vi "CRYO_MASTER_FULL_RUN2.vi"() -> ()   [LabVIEW 2017] (continued)
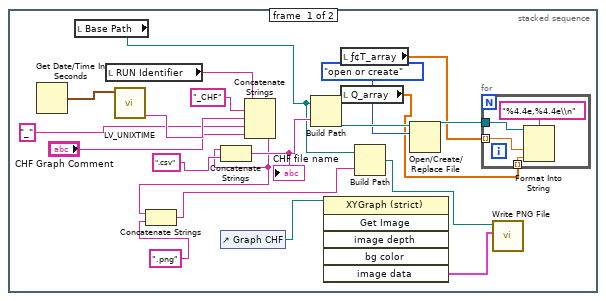
[diagram p3: hidden frame]
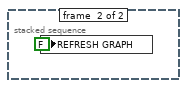
[diagram p5: hidden frame]
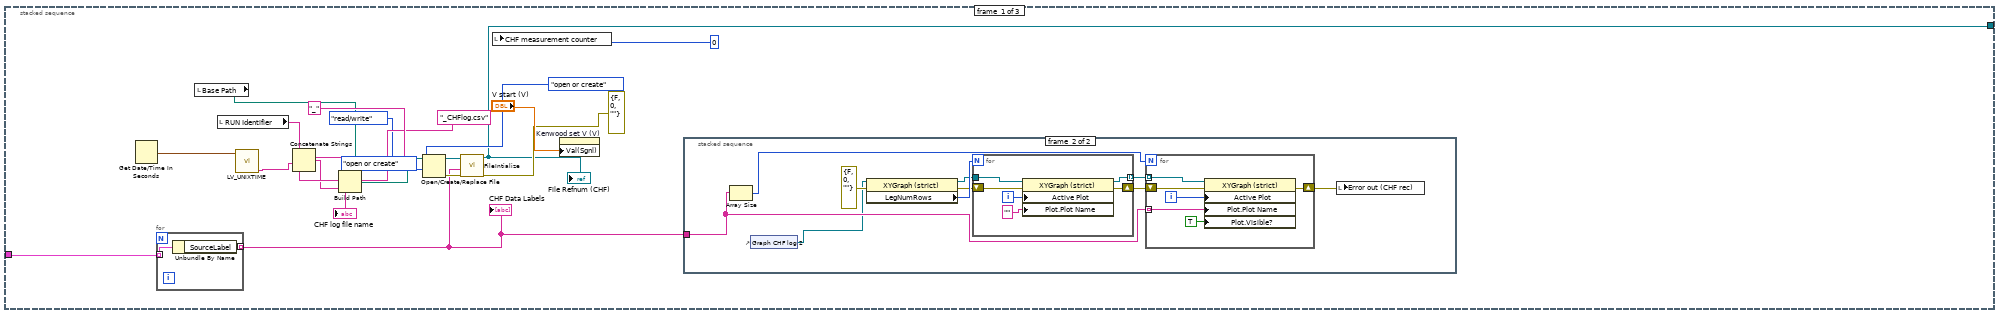
[diagram p7: hidden frame]
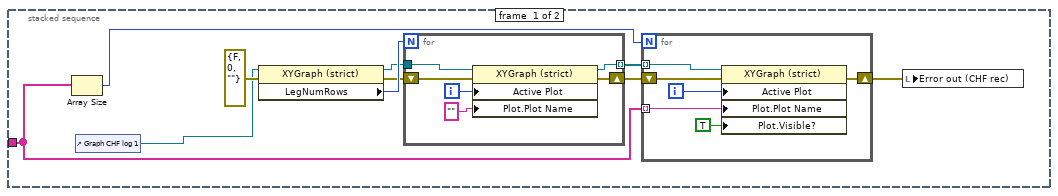
[diagram p8: hidden frame]
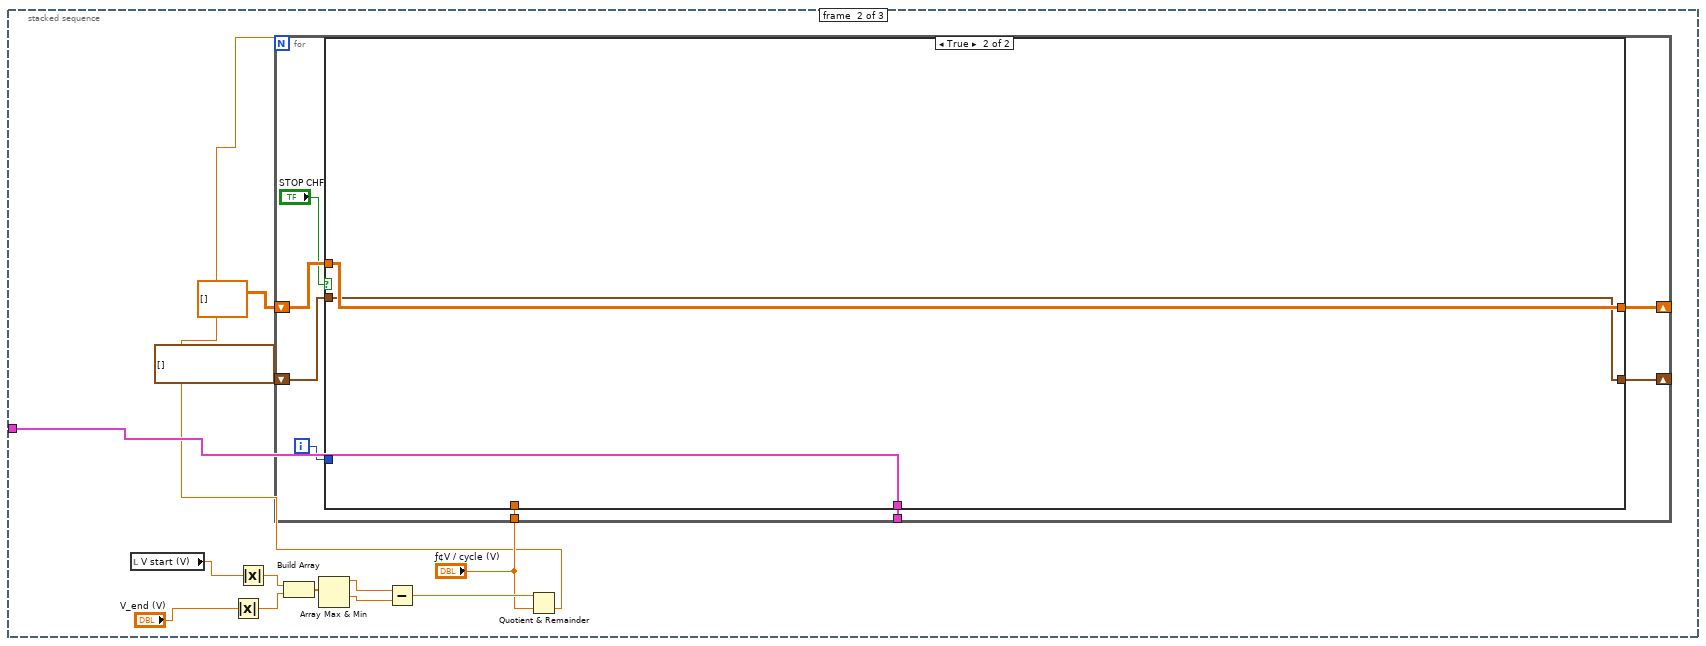
[diagram p9: hidden frame]
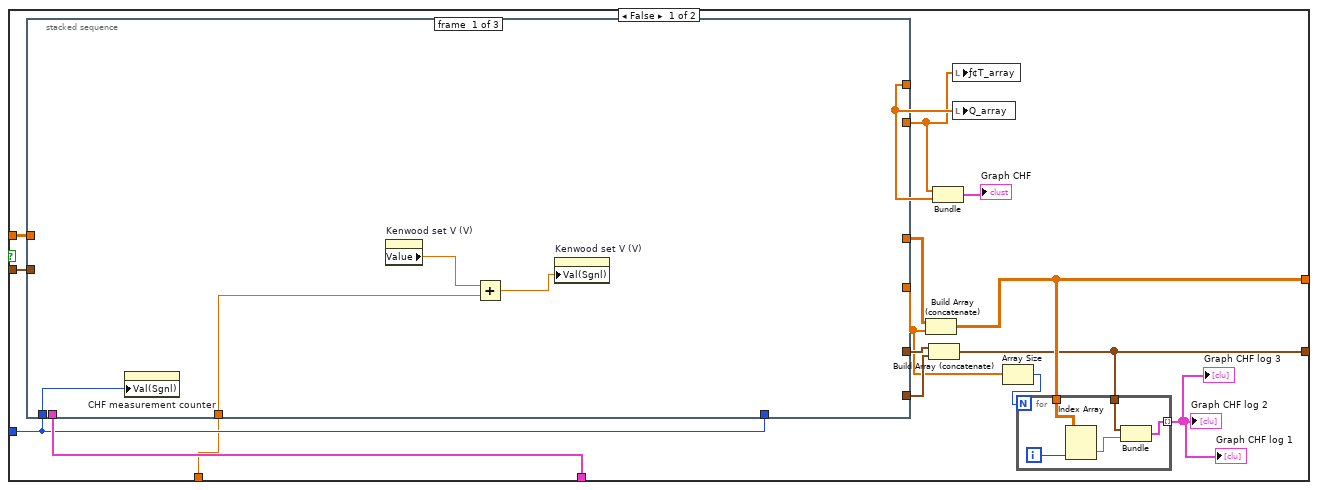
[diagram p10: hidden frame]
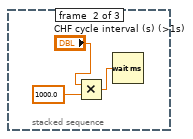
[diagram p11: hidden frame]
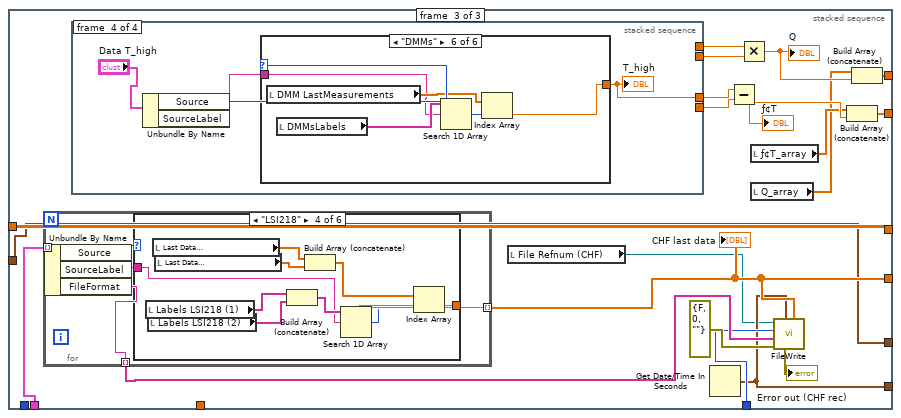
[diagram p12: hidden frame]
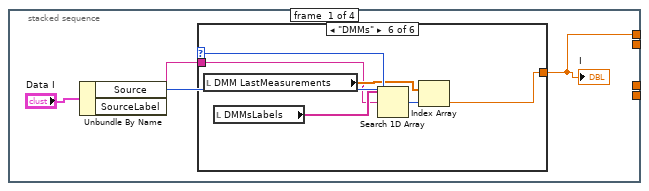
[diagram p13: hidden frame]
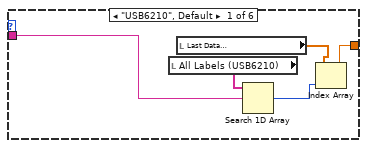
[diagram p14: hidden frame]
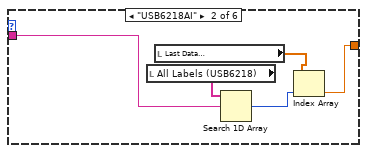
[diagram p15: hidden frame]
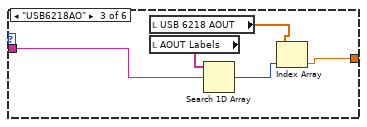
[diagram p16: hidden frame]
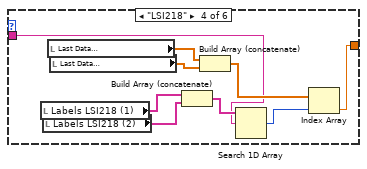
[diagram p17: hidden frame]
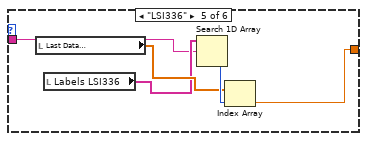
[diagram p18: hidden frame]
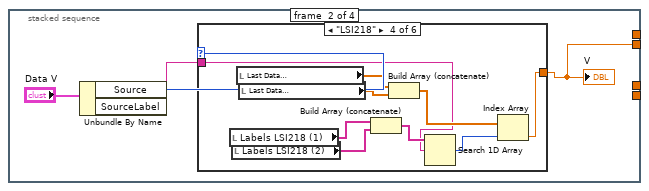
[diagram p19: hidden frame]
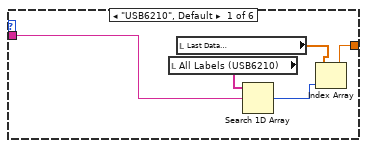
[diagram p20: hidden frame]
            n999 = for {
              tunnel: w2038 -> [w2050]
              tunnel: w2037 -> [w2048] mode=indexing
              tunnel: w2036 -> [w2047] mode=indexing
              n1000 = Format Into String(format string="%4.4e,%4.4e\\n" ("prompt"), initial string=w2050, w2048, w2047) -> ()  [unwired: 1 in, 2 out]
            }
            n1001 = call <vilib>:"Write PNG File.vi"("image data"=w2027, "path to PNG file"=w2028) -> ()  [unwired: 8 in, 2 out]
          }
          frame #1 {
            n1002 = local write "RECORD GRAPH"(FALSE ("RECORD GRAPH")) -> ()
          }
        }
      }
    }
    n1003 = case shown="True" "START CHF" {
      tunnel: "RecordSettings" -> [_ w2055]
      frame False {
      }
      frame True {
        n1004 = stacked-sequence {
          tunnel: [w2059 _ _] -> _
          tunnel: w2055 -> [w2058 w2132 _]
          frame #0 {
            (unwired) T24."open or create" ("operation (0:open)")
            n1005 = Get Date/Time In Seconds() -> (seconds since 1Jan1904=w2071:timestamp)
            n1006 = for {
              tunnel: [w2119] -> w2057 mode=indexing
              tunnel: w2058 -> [w2118] mode=indexing
              n1007 = Unbundle By Name(w2118) -> ("SourceLabel"=w2119:string)
            }
            "CHF Data Labels" <- w2057
            n1008 = local read "Base Path"() -> (w2066:path)
            n1009 = local read "RUN Identifier"() -> (w2070:string)
            n1010 = call "LV_UNIXTIME.vi"("current time"=w2071) -> ("date/time string"=w2069:string)  [unwired: 9 in, 1 out]
            n1011 = Concatenate Strings(w2070, "_" ("string"), w2069, "_CHFlog.csv" ("string")) -> (w2065:string)
            "CHF log file name" <- w2065
            n1012 = Build Path(base path=w2066, name or relative path=w2065) -> (appended path=w2064:path)
            n1013 = Open/Create/Replace File(file path (use dialog)=w2064, error in=errorcluster {"status"=FALSE, "code"=0, "source"=""}, operation (0:open)=T24."open or create", access (0:read/write)=enum16{"read/write", "read-only", "write-only"}."read/write") -> (refnum out=w2062:refnum<file>, error out=w2061:errorcluster)  [unwired: 2 in, 1 out]
            n1014 = call "FileIntialize.vi"("Error In"=w2061, "Labels"=w2057, "refnum in"=w2062) -> ("File Refnum"=w2059:refnum<file>)  [unwired: 7 in, 1 out]
            "File Refnum (CHF)" <- w2059
            n1015 = local write "CHF measurement counter"(0 ("CHF counter")) -> ()
            n1016 = property on="Kenwood set V (V)" class="DigNum (strict)"("Val(Sgnl)"="V start (V)") -> ()  [unwired: 2 in, 2 out]
            n1017 = stacked-sequence {
              tunnel: w2057 -> [w2075 w2098]
              frame #0 {
                n1018 = Array Size(array=w2075) -> (size(s)=w2083:i32)
                n1019 = control-ref of="Graph CHF log 1"() -> (w2076:refnum<vi>)
                n1020 = property class="XYGraph (strict)"(reference=w2076, error in=errorcluster {"status"=FALSE, "code"=0, "source"=""} ("error in (no error)")) -> (reference out=w2078:refnum<vi>, error out=w2080:errorcluster, "LegNumRows"=w2081:u32)
                n1021 = for {
                  N: w2081 -> [_]
                  shift-right: [w2092] -> w2082
                  shift-left: w2080 -> [w2093]
                  tunnel: w2078 -> [w2091]
                  tunnel: [w2090] -> w2077 mode=indexing
                  i -> [w2095]
                  n1022 = property class="XYGraph (strict)"(reference=w2091, error in=w2093, "Active Plot"=w2095, "Plot.Plot Name"="") -> (reference out=w2090:refnum<vi>, error out=w2092:errorcluster)
                }
                n1023 = for {
                  N: w2083 -> [_]
                  shift-right: [w2087] -> w2074
                  shift-left: w2082 -> [w2088]
                  tunnel: w2077 -> [w2085] mode=indexing
                  tunnel: w2075 -> [w2084] mode=indexing
                  i -> [w2089]
                  n1024 = property class="XYGraph (strict)"(reference=w2085, error in=w2088, "Active Plot"=w2089, "Plot.Plot Name"=w2084, "Plot.Visible?"=TRUE ("Plot.Visible")) -> (error out=w2087:errorcluster)  [unwired: 1 out]
                }
                n1025 = local write "Error out (CHF rec)"(w2074) -> ()
              }
              frame #1 {
                n1026 = Array Size(array=w2098) -> (size(s)=w2105:i32)
                n1027 = control-ref of="Graph CHF log 2"() -> (w2097:refnum<vi>)
                n1028 = property class="XYGraph (strict)"(reference=w2097, error in=errorcluster {"status"=FALSE, "code"=0, "source"=""} ("error in (no error)")) -> (reference out=w2100:refnum<vi>, error out=w2102:errorcluster, "LegNumRows"=w2103:u32)
                n1029 = for {
                  N: w2103 -> [_]
                  shift-right: [w2114] -> w2104
                  shift-left: w2102 -> [w2115]
                  tunnel: w2100 -> [w2113]
                  tunnel: [w2112] -> w2099 mode=indexing
                  i -> [w2117]
                  n1030 = property class="XYGraph (strict)"(reference=w2113, error in=w2115, "Active Plot"=w2117, "Plot.Plot Name"="") -> (reference out=w2112:refnum<vi>, error out=w2114:errorcluster)
                }
                n1031 = for {
                  N: w2105 -> [_]
                  shift-right: [w2109] -> w2096
                  shift-left: w2104 -> [w2110]
                  tunnel: w2099 -> [w2107] mode=indexing
                  tunnel: w2098 -> [w2106] mode=indexing
                  i -> [w2111]
                  n1032 = property class="XYGraph (strict)"(reference=w2107, error in=w2110, "Active Plot"=w2111, "Plot.Plot Name"=w2106, "Plot.Visible?"=TRUE ("Plot.Visible")) -> (error out=w2109:errorcluster)  [unwired: 1 out]
                }
                n1033 = local write "Error out (CHF rec)"(w2096) -> ()
              }
            }
          }
          frame #1 {
            n1034 = local read "V start (V)"() -> (w2131:dbl)
            n1035 = Absolute Value(x="V_end (V)") -> (abs(x)=w2128:dbl)
            n1036 = Absolute Value(x=w2131) -> (abs(x)=w2129:dbl)
            n1037 = Build Array(w2129, w2128) -> (w2127:dbl[])
            n1038 = Array Max & Min(array=w2127) -> (max value=w2126:dbl, min value=w2125:dbl)  [unwired: 2 out]
            n1039 = Subtract(x=w2126, y=w2125) -> (x-y=w2124:dbl)
            n1040 = Quotient & Remainder(x=w2124, y="ƒ¢V / cycle (V)") -> (floor(x/y)=w2122:dbl)  [unwired: 1 out]
            n1041 = for {
              N: w2122 -> [_]
              tunnel: w2132 -> [w2140]
              shift-right: [w2136] -> _
              shift-left: dbl[][] [] -> [w2138]
              shift-right: [w2135] -> _
              shift-left: timestamp[] [] -> [w2137]
              tunnel: "ƒ¢V / cycle (V)" -> [w2134]
              i -> [w2139]
              n1042 = case shown="True" "STOP CHF" {
                tunnel: w2140 -> [w2156 _]
                tunnel: w2139 -> [w2155 _]
                tunnel: w2138 -> [w2154 w2381]
                tunnel: w2137 -> [w2150 w2380]
                tunnel: [w2147 w2381] -> w2136
                tunnel: [w2146 w2380] -> w2135
                tunnel: w2134 -> [w2141 _]
                frame False {
                  n1043 = stacked-sequence {
                    tunnel: w2156 -> [_ _ w2188]
                    tunnel: [_ _ w2179] -> w2145
                    tunnel: w2155 -> [_ _ w2178]
                    tunnel: w2155 -> [w2163 _ _]
                    tunnel: [_ _ w2176] -> w2144
                    tunnel: [_ _ w2175] -> w2149
                    tunnel: [_ _ w2174] -> w2153
                    tunnel: w2154 -> [_ _ w2174]
                    tunnel: [_ _ w2173] -> w2152
                    tunnel: w2150 -> [_ _ w2172]
                    tunnel: [_ _ w2172] -> w2151
                    tunnel: w2141 -> [w2162 _ _]
                    frame #0 {
                      n1044 = property on="CHF measurement counter" class="DigNum (strict)"("Val(Sgnl)"=w2163) -> ()  [unwired: 2 in, 2 out]
                      n1045 = property on="Kenwood set V (V)" class="DigNum (strict)"() -> ("Value"=w2165:dbl)  [unwired: 2 in, 2 out]
                      n1046 = Add(x=w2165, y=w2162) -> (x+y=w2164:dbl)
                      n1047 = property on="Kenwood set V (V)" class="DigNum (strict)"("Val(Sgnl)"=w2164) -> ()  [unwired: 2 in, 2 out]
                    }
                    frame #1 {
                      n1048 = Multiply(x="CHF cycle interval (s) (>1s)", y=1000.0) -> (x*y=w2167:dbl)
                      n1049 = Wait (ms)(milliseconds to wait=w2167) -> ()  [unwired: 1 out]
                    }
                    frame #2 {
                      n1050 = for {
                        tunnel: w2188 -> [w2345] mode=indexing
                        tunnel: [w2343] -> w2175 mode=indexing
                        tunnel: [w2341] -> w2186 mode=indexing
                        n1051 = Unbundle By Name(w2345) -> ("Source"=w2344:T34, "SourceLabel"=w2342:string, "FileFormat"=w2341:string)
                        n1052 = case shown="\"LSI218\"" w2344 {
                          tunnel: [w2346 w2351 w2356 w2362 w2370 w2375] -> w2343
                          tunnel: w2342 -> [w2347 w2353 w2358 w2361 w2371 w2379]
                          frame "USB6210", Default {
                            n1053 = local read "All Labels (USB6210)"() -> (w2349:string[])
                            n1054 = local read "Last Data \n(USB6210)"() -> (w2350:dbl[])
                            n1055 = Search 1D Array(1D array=w2349, element=w2347) -> (index of element=w2348:i32)  [unwired: 1 in]
                            n1056 = Index Array(array=w2350, index=w2348) -> (element=w2346:dbl)
                          }
                          frame "USB6218AI" {
                            n1057 = local read "All Labels (USB6218)"() -> (w2354:string[])
                            n1058 = local read "Last Data \n(USB6218)"() -> (w2355:dbl[])
                            n1059 = Search 1D Array(1D array=w2354, element=w2353) -> (index of element=w2352:i32)  [unwired: 1 in]
                            n1060 = Index Array(array=w2355, index=w2352) -> (element=w2351:dbl)
                          }
                          frame "USB6218AO" {
                            n1061 = local read "USB 6218 AOUT"() -> (w2360:dbl[])
                            n1062 = local read "AOUT Labels"() -> (w2359:string[])
                            n1063 = Search 1D Array(1D array=w2359, element=w2358) -> (index of element=w2357:i32)  [unwired: 1 in]
                            n1064 = Index Array(array=w2360, index=w2357) -> (element=w2356:dbl)
                          }
                          frame "LSI218" {
                            n1065 = local read "Labels LSI218 (1)"() -> (w2365:string[])
                            n1066 = local read "Labels LSI218 (2)"() -> (w2364:string[])
                            n1067 = local read "Last Data \nLSI218 (1)"() -> (w2368:dbl[])
                            n1068 = local read "Last Data \nLSI218 (2)"() -> (w2367:dbl[])
                            n1069 = Build Array (concatenate)(w2365, w2364) -> (w2363:string[])
                            n1070 = Build Array (concatenate)(w2368, w2367) -> (w2366:dbl[])
                            n1071 = Search 1D Array(1D array=w2363, element=w2361) -> (index of element=w2369:i32)  [unwired: 1 in]
                            n1072 = Index Array(array=w2366, index=w2369) -> (element=w2362:dbl)
                          }
                          frame "LSI336" {
                            n1073 = local read "Last Data \nLSI336"() -> (w2373:dbl[])
                            n1074 = local read "Labels LSI336"() -> (w2374:string[])
                            n1075 = Search 1D Array(1D array=w2374, element=w2371) -> (index of element=w2372:i32)  [unwired: 1 in]
                            n1076 = Index Array(array=w2373, index=w2372) -> (element=w2370:dbl)
                          }
                          frame "DMMs" {
                            n1077 = local read "DMM LastMeasurements"() -> (w2376:dbl[])
                            n1078 = local read "DMMsLabels"() -> (w2378:string[])
                            n1079 = Search 1D Array(1D array=w2378, element=w2379) -> (index of element=w2377:i32)  [unwired: 1 in]
                            n1080 = Index Array(array=w2376, index=w2377) -> (element=w2375:dbl)
                          }
                        }
                      }
                      "CHF last data" <- w2175
                      n1081 = stacked-sequence {
                        tunnel: [w2189 _ _ _] -> w2184
                        tunnel: [_ w2227 _ _] -> w2183
                        tunnel: [_ _ _ w2303] -> w2182
                        tunnel: [_ _ w2265 _] -> w2181
                        frame #0 {
                          n1082 = Unbundle By Name("Data I") -> ("Source"=w2191:T34, "SourceLabel"=w2190:string)
                          n1083 = case shown="\"DMMs\"" w2191 {
                            tunnel: w2190 -> [w2194 w2199 w2204 w2209 w2218 w2223]
                            tunnel: [w2193 w2198 w2203 w2208 w2217 w2222] -> w2189
                            frame "USB6210", Default {
                              n1084 = local read "All Labels (USB6210)"() -> (w2196:string[])
                              n1085 = local read "Last Data \n(USB6210)"() -> (w2195:dbl[])
                              n1086 = Search 1D Array(1D array=w2196, element=w2194) -> (index of element=w2197:i32)  [unwired: 1 in]
                              n1087 = Index Array(array=w2195, index=w2197) -> (element=w2193:dbl)
                            }
                            frame "USB6218AI" {
                              n1088 = local read "All Labels (USB6218)"() -> (w2201:string[])
                              n1089 = local read "Last Data \n(USB6218)"() -> (w2200:dbl[])
                              n1090 = Search 1D Array(1D array=w2201, element=w2199) -> (index of element=w2202:i32)  [unwired: 1 in]
                              n1091 = Index Array(array=w2200, index=w2202) -> (element=w2198:dbl)
                            }
                            frame "USB6218AO" {
                              n1092 = local read "USB 6218 AOUT"() -> (w2205:dbl[])
                              n1093 = local read "AOUT Labels"() -> (w2206:string[])
                              n1094 = Search 1D Array(1D array=w2206, element=w2204) -> (index of element=w2207:i32)  [unwired: 1 in]
                              n1095 = Index Array(array=w2205, index=w2207) -> (element=w2203:dbl)
                            }
                            frame "LSI218" {
                              n1096 = local read "Labels LSI218 (1)"() -> (w2214:string[])
                              n1097 = local read "Labels LSI218 (2)"() -> (w2215:string[])
                              n1098 = local read "Last Data \nLSI218 (1)"() -> (w2211:dbl[])
                              n1099 = local read "Last Data \nLSI218 (2)"() -> (w2212:dbl[])
                              n1100 = Build Array (concatenate)(w2214, w2215) -> (w2216:string[])
                              n1101 = Build Array (concatenate)(w2211, w2212) -> (w2213:dbl[])
                              n1102 = Search 1D Array(1D array=w2216, element=w2209) -> (index of element=w2210:i32)  [unwired: 1 in]
                              n1103 = Index Array(array=w2213, index=w2210) -> (element=w2208:dbl)
                            }
                            frame "LSI336" {
                              n1104 = local read "Last Data \nLSI336"() -> (w2220:dbl[])
                              n1105 = local read "Labels LSI336"() -> (w2219:string[])
                              n1106 = Search 1D Array(1D array=w2219, element=w2218) -> (index of element=w2221:i32)  [unwired: 1 in]
                              n1107 = Index Array(array=w2220, index=w2221) -> (element=w2217:dbl)
                            }
                            frame "DMMs" {
                              n1108 = local read "DMM LastMeasurements"() -> (w2226:dbl[])
                              n1109 = local read "DMMsLabels"() -> (w2224:string[])
                              n1110 = Search 1D Array(1D array=w2224, element=w2223) -> (index of element=w2225:i32)  [unwired: 1 in]
                              n1111 = Index Array(array=w2226, index=w2225) -> (element=w2222:dbl)
                            }
                          }
                          "I" <- w2189
                        }
                        frame #1 {
                          n1112 = Unbundle By Name("Data V") -> ("Source"=w2230:T34, "SourceLabel"=w2229:string)
                          n1113 = case shown="\"LSI218\"" w2230 {
                            tunnel: w2229 -> [w2232 w2237 w2242 w2247 w2256 w2261]
                            tunnel: [w2231 w2236 w2241 w2246 w2255 w2260] -> w2227
                            frame "USB6210", Default {
                              n1114 = local read "All Labels (USB6210)"() -> (w2234:string[])
                              n1115 = local read "Last Data \n(USB6210)"() -> (w2233:dbl[])
                              n1116 = Search 1D Array(1D array=w2234, element=w2232) -> (index of element=w2235:i32)  [unwired: 1 in]
                              n1117 = Index Array(array=w2233, index=w2235) -> (element=w2231:dbl)
                            }
                            frame "USB6218AI" {
                              n1118 = local read "All Labels (USB6218)"() -> (w2239:string[])
                              n1119 = local read "Last Data \n(USB6218)"() -> (w2238:dbl[])
                              n1120 = Search 1D Array(1D array=w2239, element=w2237) -> (index of element=w2240:i32)  [unwired: 1 in]
                              n1121 = Index Array(array=w2238, index=w2240) -> (element=w2236:dbl)
                            }
                            frame "USB6218AO" {
                              n1122 = local read "USB 6218 AOUT"() -> (w2243:dbl[])
                              n1123 = local read "AOUT Labels"() -> (w2244:string[])
                              n1124 = Search 1D Array(1D array=w2244, element=w2242) -> (index of element=w2245:i32)  [unwired: 1 in]
                              n1125 = Index Array(array=w2243, index=w2245) -> (element=w2241:dbl)
                            }
                            frame "LSI218" {
                              n1126 = local read "Labels LSI218 (1)"() -> (w2252:string[])
                              n1127 = local read "Labels LSI218 (2)"() -> (w2253:string[])
                              n1128 = local read "Last Data \nLSI218 (1)"() -> (w2249:dbl[])
                              n1129 = local read "Last Data \nLSI218 (2)"() -> (w2250:dbl[])
                              n1130 = Build Array (concatenate)(w2252, w2253) -> (w2254:string[])
                              n1131 = Build Array (concatenate)(w2249, w2250) -> (w2251:dbl[])
                              n1132 = Search 1D Array(1D array=w2254, element=w2247) -> (index of element=w2248:i32)  [unwired: 1 in]
                              n1133 = Index Array(array=w2251, index=w2248) -> (element=w2246:dbl)
                            }
                            frame "LSI336" {
                              n1134 = local read "Last Data \nLSI336"() -> (w2258:dbl[])
                              n1135 = local read "Labels LSI336"() -> (w2257:string[])
                              n1136 = Search 1D Array(1D array=w2257, element=w2256) -> (index of element=w2259:i32)  [unwired: 1 in]
                              n1137 = Index Array(array=w2258, index=w2259) -> (element=w2255:dbl)
                            }
                            frame "DMMs" {
                              n1138 = local read "DMM LastMeasurements"() -> (w2264:dbl[])
                              n1139 = local read "DMMsLabels"() -> (w2262:string[])
                              n1140 = Search 1D Array(1D array=w2262, element=w2261) -> (index of element=w2263:i32)  [unwired: 1 in]
                              n1141 = Index Array(array=w2264, index=w2263) -> (element=w2260:dbl)
                            }
                          }
                          "V" <- w2227
                        }
                        frame #2 {
                          n1142 = Unbundle By Name("Data T_low") -> ("Source"=w2268:T34, "SourceLabel"=w2267:string)
                          n1143 = case shown="\"DMMs\"" w2268 {
                            tunnel: w2267 -> [w2270 w2275 w2280 w2285 w2294 w2299]
                            tunnel: [w2269 w2274 w2279 w2284 w2293 w2298] -> w2265
                            frame "USB6210", Default {
                              n1144 = local read "All Labels (USB6210)"() -> (w2272:string[])
                              n1145 = local read "Last Data \n(USB6210)"() -> (w2271:dbl[])
                              n1146 = Search 1D Array(1D array=w2272, element=w2270) -> (index of element=w2273:i32)  [unwired: 1 in]
                              n1147 = Index Array(array=w2271, index=w2273) -> (element=w2269:dbl)
                            }
                            frame "USB6218AI" {
                              n1148 = local read "All Labels (USB6218)"() -> (w2277:string[])
                              n1149 = local read "Last Data \n(USB6218)"() -> (w2276:dbl[])
                              n1150 = Search 1D Array(1D array=w2277, element=w2275) -> (index of element=w2278:i32)  [unwired: 1 in]
                              n1151 = Index Array(array=w2276, index=w2278) -> (element=w2274:dbl)
                            }
                            frame "USB6218AO" {
                              n1152 = local read "USB 6218 AOUT"() -> (w2281:dbl[])
                              n1153 = local read "AOUT Labels"() -> (w2282:string[])
                              n1154 = Search 1D Array(1D array=w2282, element=w2280) -> (index of element=w2283:i32)  [unwired: 1 in]
                              n1155 = Index Array(array=w2281, index=w2283) -> (element=w2279:dbl)
                            }
                            frame "LSI218" {
                              n1156 = local read "Labels LSI218 (1)"() -> (w2290:string[])
                              n1157 = local read "Labels LSI218 (2)"() -> (w2291:string[])
                              n1158 = local read "Last Data \nLSI218 (1)"() -> (w2287:dbl[])
                              n1159 = local read "Last Data \nLSI218 (2)"() -> (w2288:dbl[])
                              n1160 = Build Array (concatenate)(w2290, w2291) -> (w2292:string[])
                              n1161 = Build Array (concatenate)(w2287, w2288) -> (w2289:dbl[])
                              n1162 = Search 1D Array(1D array=w2292, element=w2285) -> (index of element=w2286:i32)  [unwired: 1 in]
                              n1163 = Index Array(array=w2289, index=w2286) -> (element=w2284:dbl)
                            }
                            frame "LSI336" {
                              n1164 = local read "Last Data \nLSI336"() -> (w2296:dbl[])
                              n1165 = local read "Labels LSI336"() -> (w2295:string[])
                              n1166 = Search 1D Array(1D array=w2295, element=w2294) -> (index of element=w2297:i32)  [unwired: 1 in]
                              n1167 = Index Array(array=w2296, index=w2297) -> (element=w2293:dbl)
                            }
                            frame "DMMs" {
                              n1168 = local read "DMM LastMeasurements"() -> (w2302:dbl[])
                              n1169 = local read "DMMsLabels"() -> (w2300:string[])
                              n1170 = Search 1D Array(1D array=w2300, element=w2299) -> (index of element=w2301:i32)  [unwired: 1 in]
                              n1171 = Index Array(array=w2302, index=w2301) -> (element=w2298:dbl)
                            }
                          }
                          "T_low" <- w2265
                        }
                        frame #3 {
                          n1172 = Unbundle By Name("Data T_high") -> ("Source"=w2306:T34, "SourceLabel"=w2305:string)
                          n1173 = case shown="\"DMMs\"" w2306 {
                            tunnel: w2305 -> [w2308 w2313 w2318 w2323 w2332 w2337]
                            tunnel: [w2307 w2312 w2317 w2322 w2331 w2336] -> w2303
                            frame "USB6210", Default {
                              n1174 = local read "All Labels (USB6210)"() -> (w2310:string[])
                              n1175 = local read "Last Data \n(USB6210)"() -> (w2309:dbl[])
                              n1176 = Search 1D Array(1D array=w2310, element=w2308) -> (index of element=w2311:i32)  [unwired: 1 in]
                              n1177 = Index Array(array=w2309, index=w2311) -> (element=w2307:dbl)
                            }
                            frame "USB6218AI" {
                              n1178 = local read "All Labels (USB6218)"() -> (w2315:string[])
                              n1179 = local read "Last Data \n(USB6218)"() -> (w2314:dbl[])
                              n1180 = Search 1D Array(1D array=w2315, element=w2313) -> (index of element=w2316:i32)  [unwired: 1 in]
                              n1181 = Index Array(array=w2314, index=w2316) -> (element=w2312:dbl)
                            }
                            frame "USB6218AO" {
                              n1182 = local read "USB 6218 AOUT"() -> (w2319:dbl[])
                              n1183 = local read "AOUT Labels"() -> (w2320:string[])
                              n1184 = Search 1D Array(1D array=w2320, element=w2318) -> (index of element=w2321:i32)  [unwired: 1 in]
                              n1185 = Index Array(array=w2319, index=w2321) -> (element=w2317:dbl)
                            }
                            frame "LSI218" {
                              n1186 = local read "Labels LSI218 (1)"() -> (w2328:string[])
                              n1187 = local read "Labels LSI218 (2)"() -> (w2329:string[])
                              n1188 = local read "Last Data \nLSI218 (1)"() -> (w2325:dbl[])
                              n1189 = local read "Last Data \nLSI218 (2)"() -> (w2326:dbl[])
                              n1190 = Build Array (concatenate)(w2328, w2329) -> (w2330:string[])
                              n1191 = Build Array (concatenate)(w2325, w2326) -> (w2327:dbl[])
                              n1192 = Search 1D Array(1D array=w2330, element=w2323) -> (index of element=w2324:i32)  [unwired: 1 in]
                              n1193 = Index Array(array=w2327, index=w2324) -> (element=w2322:dbl)
                            }
                            frame "LSI336" {
                              n1194 = local read "Last Data \nLSI336"() -> (w2334:dbl[])
                              n1195 = local read "Labels LSI336"() -> (w2333:string[])
                              n1196 = Search 1D Array(1D array=w2333, element=w2332) -> (index of element=w2335:i32)  [unwired: 1 in]
                              n1197 = Index Array(array=w2334, index=w2335) -> (element=w2331:dbl)
                            }
                            frame "DMMs" {
                              n1198 = local read "DMM LastMeasurements"() -> (w2340:dbl[])
                              n1199 = local read "DMMsLabels"() -> (w2338:string[])
                              n1200 = Search 1D Array(1D array=w2338, element=w2337) -> (index of element=w2339:i32)  [unwired: 1 in]
                              n1201 = Index Array(array=w2340, index=w2339) -> (element=w2336:dbl)
                            }
                          }
                          "T_high" <- w2303
                        }
                      }
                      n1202 = local read "File Refnum (CHF)"() -> (w2169:refnum<file>)
                      n1203 = Get Date/Time In Seconds() -> (seconds since 1Jan1904=w2173:timestamp)
                      n1204 = Subtract(x=w2182, y=w2181) -> (x-y=w2177:dbl)
                      "ƒ¢T" <- w2177
                      n1205 = Multiply(x=w2184, y=w2183) -> (x*y=w2180:dbl)
                      "Q" <- w2180
                      n1206 = local read "ƒ¢T_array"() -> (w2171:dbl[])
                      n1207 = local read "Q_array"() -> (w2170:dbl[])
                      n1208 = call "FileWrite.vi"("DataArray"=w2175, "Time Stamp"=w2173, "Error In"=errorcluster {"status"=FALSE, "code"=0, "source"=""}, "FileFormat"=w2186, "Index"=w2178, "refnum in"=w2169) -> ("Error Out"=→"Error out (CHF rec)":errorcluster)  [unwired: 4 in, 1 out]
                      n1209 = Build Array (concatenate)(w2171, w2177) -> (w2176:dbl[])
                      n1210 = Build Array (concatenate)(w2170, w2180) -> (w2179:dbl[])
                    }
                  }
                  n1211 = Build Array (concatenate)(w2153, w2149) -> (w2147:dbl[][])
                  n1212 = Build Array (concatenate)(w2151, w2152) -> (w2146:timestamp[])
                  n1213 = Bundle(w2144, w2145) -> (→"Graph CHF":cluster{dbl[], dbl[]})  [unwired: 1 in]
                  n1214 = local write "ƒ¢T_array"(w2144) -> ()
                  n1215 = local write "Q_array"(w2145) -> ()
                  n1216 = Array Size(array=w2149) -> (size(s)=w2148:i32)
                  n1217 = for {
                    N: w2148 -> [_]
                    tunnel: w2147 -> [w2161]
                    tunnel: w2146 -> [w2159]
                    tunnel: [w2157] -> w2142 mode=indexing
                    i -> [w2160]
                    n1218 = Index Array(array=w2161, index (col)=w2160) -> (element=w2158:dbl[])  [unwired: 1 in]
                    n1219 = Bundle(w2159, w2158) -> (w2157:cluster{timestamp[], dbl[]})  [unwired: 1 in]
                  }
                  "Graph CHF log 2" <- w2142
                  "Graph CHF log 1" <- w2142
                  "Graph CHF log 3" <- w2142
                }
                frame True {
                }
              }
            }
          }
          frame #2 {
            n1220 = local write "CHF measurement counter"(0 ("CHF counter")) -> ()
            n1221 = local write "START CHF"(FALSE ("START CHF")) -> ()
            n1222 = local write "STOP CHF"(FALSE ("STOP CHF")) -> ()
          }
        }
      }
    }
    n1223 = case shown="True" "REFRESH GRAPH" {
      frame False {
      }
      frame True {
        n1224 = stacked-sequence {
          frame #0 {
            w2053 = dbl[] [] ("ƒ¢T_array")
            n1225 = local write "ƒ¢T_array"(w2053) -> ()
            n1226 = local write "Q_array"(w2053) -> ()
            n1227 = Bundle("ƒ¢T_array"=w2053, "ƒ¢T_array"=w2053) -> (w2052:cluster{"ƒ¢T_array":dbl[], "ƒ¢T_array":dbl[]})  [unwired: 1 in]
            n1228 = local write "Graph CHF"(w2052) -> ()
          }
          frame #1 {
            n1229 = local write "REFRESH GRAPH"(FALSE ("REFRESH GRAPH")) -> ()
          }
        }
      }
    }
    n1230 = Get Notifier Status(notifier=w2022, error in (no error)=w2021) -> (current notification=w2023:bool)  [unwired: 4 out]
  }
  n1231 = while {
    shift-right: [w2394] -> w6
    shift-left: refnum<class "DMMsData.lvclass"> refnum ("DMMsData.lvclass") -> [w2393]
    shift-right: [w2392] -> w5
    shift-left: errorcluster {"status"=FALSE, "code"=0, "source"=""} ("error in (no error)") -> [w2385]
    tunnel: w3 -> [w2390]
    tunnel: w2 -> [w2389]
    tunnel: [w2388] -> w9
    i -> [w2391]
    stop <- w2387 stop-if-true
    n1232 = Equal?(x=w2391, y=0) -> (x = y?=w2395:bool)
    n1233 = Wait (ms)(milliseconds to wait="Measurement Interval DMMs (ms)") -> ()  [unwired: 1 out]
    n1234 = case shown="True" "Measure DMMs?" {
      tunnel: w2395 -> [_ w2406]
      tunnel: [w2399 w2404] -> w2394
      tunnel: w2393 -> [w2399 w2403]
      tunnel: w2385 -> [w2398 w2402]
      tunnel: [w2398 w2401] -> w2392
      tunnel: w2391 -> [_ w2400]
      frame False {
      }
      frame True {
        n1235 = Or(x="Initialize (DMMs)", y=w2406) -> (x .or. y?=w2405:bool)
        n1236 = case shown="True" w2405 {
          tunnel: w2403 -> [w2437 w2473]
          tunnel: [w2434 w2472] -> w2404
          tunnel: w2402 -> [w2436 w2469]
          tunnel: [w2435 w2466] -> w2401
          tunnel: w2400 -> [w2433 _]
          frame False {
            n1237 = local read "VariableSources"() -> (w2426:T11)
            n1238 = for {
              tunnel: w2426 -> [w2440] mode=indexing
              tunnel: [w2439] -> w2425 mode=indexing
              tunnel: [w2438] -> w2424 mode=indexing
              n1239 = case shown="\"LSI218\"" w2440 {
                tunnel: [w2442 w2444 w2446 w2447 w2453] -> w2439
                tunnel: [w2441 w2443 w2445 w2448 w2454] -> w2438
                frame "USB6210" {
                  n1240 = local read "All Labels (USB6210)"() -> (w2442:string[])
                  n1241 = local read "Last Data \n(USB6210)"() -> (w2441:dbl[])
                }
                frame "USB6218AI" {
                  n1242 = local read "Last Data \n(USB6218)"() -> (w2443:dbl[])
                  n1243 = local read "All Labels (USB6218)"() -> (w2444:string[])
                }
                frame "USB6218AO" {
                  n1244 = local read "USB 6218 AOUT"() -> (w2445:dbl[])
                  n1245 = local read "AOUT Labels"() -> (w2446:string[])
                }
                frame "LSI218" {
                  n1246 = local read "Last Data \nLSI218 (2)"() -> (w2449:dbl[])
                  n1247 = local read "Last Data \nLSI218 (1)"() -> (w2450:dbl[])
                  n1248 = local read "Labels LSI218 (2)"() -> (w2452:string[])
                  n1249 = local read "Labels LSI218 (1)"() -> (w2451:string[])
                  n1250 = Build Array (concatenate)(w2450, w2449) -> (w2448:dbl[])
                  n1251 = Build Array (concatenate)(w2451, w2452) -> (w2447:string[])
                }
                frame "LSI336" {
                  n1252 = local read "Last Data \nLSI336"() -> (w2454:dbl[])
                  n1253 = local read "Labels LSI336"() -> (w2453:string[])
                }
              }
            }
            n1254 = local read "DMMsConfig (variables)"() -> (w2418:T12)
            n1255 = local read "DMMsConfig"() -> (w2430:T13)
            n1256 = call-dynamic "DMMs_measure.vi"("DMMsData in"=w2437, "Sample #"="Sample #", "MeasurementIndex"=w2433, "SourceDataLabels"=w2425, "error in (no error)"=w2436, "SourceDataArray"=w2424) -> ("TimeArray"=w2432:timestamp[], "DMMsData out"=w2434:refnum<class "DMMsData.lvclass">, "LastData"=w2412:dbl[], "DataArray"=w2429:dbl[][], "DeviceActive?"=→"Active?":bool[], "error out"=w2435:errorcluster)  [unwired: 4 in]
            "DMM LastMeasurements" <- w2412
            n1257 = Array Size(array=w2418) -> (size(s)=w2416:i32)
            n1258 = Array Size(array=w2430) -> (size(s)=w2417:i32)
            n1259 = Add(x=w2417, y=w2416) -> (x+y=w2415:i32)
            n1260 = for {
              N: w2415 -> [_]
              tunnel: w2432 -> [w2457]
              tunnel: w2429 -> [w2461]
              shift-right: [w2455] -> w2414
              shift-left: T4 [] -> [w2456]
              i -> [w2460]
              n1261 = Index Array(array=w2461, index (col)=w2460) -> (element=w2459:dbl[])  [unwired: 1 in]
              n1262 = Bundle("TimeArray"=w2457, "DataArray"=w2459) -> (w2458:T33)  [unwired: 1 in]
              n1263 = Build Array (concatenate)(w2456, w2458) -> (w2455:T4)
            }
            "Graph DMMs 2" <- w2414
            "Graph DMMs 1" <- w2414
            "Graph DMMs 3" <- w2414
            n1264 = Index Array(array=w2412, index #1="index T_2", index #2="index T_ 1") -> (element #1=w2411:dbl, element #2=w2408:dbl)
            n1265 = Index Array(array=w2412, index #1="index V", index #2="index I") -> (element #1=w2421:dbl, element #2=w2420:dbl)
            n1266 = Subtract(x=w2411, y=w2408) -> (x-y=→"ƒ¢T=T_2 -T_1":dbl)
            n1267 = Multiply(x=w2421, y=w2420) -> (x*y=→"Q = I *V":dbl)
          }
          frame True {
            n1268 = local write "Initialize (DMMs)"(FALSE ("Initialize 2")) -> ()
            n1269 = local read "RUN Identifier"() -> (w2464:string)
            n1270 = local read "Base Path"() -> (w2470:path)
            n1271 = call-dynamic "DMMs_initialize.vi"("DMMsConfig (variables)"="DMMsConfig (variables)", "DMMsConfig"="DMMsConfig", "InstName"="InstName DMMs", "error in (no error)"=w2469, "base path"=w2470, "RunIdentifier"=w2464, "DMMsData in"=w2473) -> ("error out"=w2466:errorcluster, "DMMsLabels"=w2467:string[], "FileName"=→"DMMFileName":string, "DMMsData out"=w2472:refnum<class "DMMsData.lvclass">, "VariableSources"=→"VariableSources":T11)
            "DMMsLabels" <- w2467
            n1272 = stacked-sequence {
              tunnel: w2467 -> [w2475 w2498 w2521]
              frame #0 {
                n1273 = Array Size(array=w2475) -> (size(s)=w2484:i32)
                n1274 = control-ref of="Graph DMMs 1"() -> (w2481:refnum<vi>)
                n1275 = property class="XYGraph (strict)"(reference=w2481, error in=errorcluster {"status"=FALSE, "code"=0, "source"=""} ("error in (no error)")) -> (reference out=w2477:refnum<vi>, error out=w2480:errorcluster, "LegNumRows"=w2482:u32)
                n1276 = for {
                  N: w2482 -> [_]
                  shift-right: [w2493] -> w2483
                  shift-left: w2480 -> [w2494]
                  tunnel: w2477 -> [w2492]
                  tunnel: [w2491] -> w2476 mode=indexing
                  i -> [w2496]
                  n1277 = property class="XYGraph (strict)"(reference=w2492, error in=w2494, "Active Plot"=w2496, "Plot.Plot Name"="") -> (reference out=w2491:refnum<vi>, error out=w2493:errorcluster)
                }
                n1278 = for {
                  N: w2484 -> [_]
                  shift-right: [w2488] -> w2478
                  shift-left: w2483 -> [w2489]
                  tunnel: w2476 -> [w2486] mode=indexing
                  tunnel: w2475 -> [w2485] mode=indexing
                  i -> [w2490]
                  n1279 = property class="XYGraph (strict)"(reference=w2486, error in=w2489, "Active Plot"=w2490, "Plot.Plot Name"=w2485, "Plot.Visible?"=TRUE ("Plot.Visible")) -> (error out=w2488:errorcluster)  [unwired: 1 out]
                }
                "error out (DMM graphs)" <- w2478
              }
              frame #1 {
                n1280 = Array Size(array=w2498) -> (size(s)=w2506:i32)
                n1281 = control-ref of="Graph DMMs 2"() -> (w2501:refnum<vi>)
                n1282 = property class="XYGraph (strict)"(reference=w2501, error in=errorcluster {"status"=FALSE, "code"=0, "source"=""} ("error in (no error)")) -> (reference out=w2500:refnum<vi>, error out=w2503:errorcluster, "LegNumRows"=w2504:u32)
                n1283 = for {
                  N: w2504 -> [_]
                  shift-right: [w2515] -> w2505
                  shift-left: w2503 -> [w2516]
                  tunnel: w2500 -> [w2514]
                  tunnel: [w2513] -> w2499 mode=indexing
                  i -> [w2518]
                  n1284 = property class="XYGraph (strict)"(reference=w2514, error in=w2516, "Active Plot"=w2518, "Plot.Plot Name"="") -> (reference out=w2513:refnum<vi>, error out=w2515:errorcluster)
                }
                n1285 = for {
                  N: w2506 -> [_]
                  shift-right: [w2510] -> w2497
                  shift-left: w2505 -> [w2511]
                  tunnel: w2499 -> [w2508] mode=indexing
                  tunnel: w2498 -> [w2507] mode=indexing
                  i -> [w2512]
                  n1286 = property class="XYGraph (strict)"(reference=w2508, error in=w2511, "Active Plot"=w2512, "Plot.Plot Name"=w2507, "Plot.Visible?"=TRUE ("Plot.Visible")) -> (error out=w2510:errorcluster)  [unwired: 1 out]
                }
                n1287 = local write "error out (DMM graphs)"(w2497) -> ()
              }
              frame #2 {
                n1288 = Array Size(array=w2521) -> (size(s)=w2528:i32)
                n1289 = control-ref of="Graph DMMs 3"() -> (w2519:refnum<vi>)
                n1290 = property class="XYGraph (strict)"(reference=w2519, error in=errorcluster {"status"=FALSE, "code"=0, "source"=""} ("error in (no error)")) -> (reference out=w2523:refnum<vi>, error out=w2525:errorcluster, "LegNumRows"=w2526:u32)
                n1291 = for {
                  N: w2526 -> [_]
                  shift-right: [w2537] -> w2527
                  shift-left: w2525 -> [w2538]
                  tunnel: w2523 -> [w2536]
                  tunnel: [w2535] -> w2522 mode=indexing
                  i -> [w2540]
                  n1292 = property class="XYGraph (strict)"(reference=w2536, error in=w2538, "Active Plot"=w2540, "Plot.Plot Name"="") -> (reference out=w2535:refnum<vi>, error out=w2537:errorcluster)
                }
                n1293 = for {
                  N: w2528 -> [_]
                  shift-right: [w2532] -> w2520
                  shift-left: w2527 -> [w2533]
                  tunnel: w2522 -> [w2530] mode=indexing
                  tunnel: w2521 -> [w2529] mode=indexing
                  i -> [w2534]
                  n1294 = property class="XYGraph (strict)"(reference=w2530, error in=w2533, "Active Plot"=w2534, "Plot.Plot Name"=w2529, "Plot.Visible?"=TRUE ("Plot.Visible")) -> (error out=w2532:errorcluster)  [unwired: 1 out]
                }
                n1295 = local write "error out (DMM graphs)"(w2520) -> ()
              }
            }
          }
        }
        "error out (DMMs)" <- w2401
      }
    }
    n1296 = Get Notifier Status(notifier=w2390, error in (no error)=w2389) -> (current notification=w2387:bool, error out=w2388:errorcluster)  [unwired: 3 out]
    "cycle # (DMMs)" <- w2391
  }
  n1297 = call-dynamic "USBData_terminate.vi"("error in (no error)"=w22, "USBData in"=w23) -> ("error out"=w24:errorcluster)  [unwired: 8 in, 1 out]
  n1298 = local write "error out (USB6210)"(w24) -> ()
  n1299 = call-dynamic "DMMs_terminate.vi"("error in (no error)"=w5, "DMMsData in"=w6) -> ("error out"=→"error out (DMMs) 2":errorcluster)  [unwired: 8 in, 1 out]
  n1300 = call-dynamic "USBData_terminate.vi"("error in (no error)"=w37, "USBData in"=w38) -> ("error out"=w39:errorcluster)  [unwired: 8 in, 1 out]
  n1301 = call-dynamic "LSI336Data_terminate.vi"("error in (no error)"=w28, "LSI336Data in"=w29) -> ("error out"=w27:errorcluster)  [unwired: 8 in, 1 out]
  n1302 = Merge Errors(w9, w11) -> (w12:errorcluster)
  n1303 = local write "error out (USB6210)"(w39) -> ()
  n1304 = local write "error out (LSI336)"(w27) -> ()
  n1305 = call "LSI218Data_terminate.vi"("error in (no error)"=w32, "LSI218Data in"=w33) -> ("error out"=w31:errorcluster)  [unwired: 8 in, 1 out]
  n1306 = Release Notifier(notifier=w10, error in (no error)=w12) -> (error out=→"error out (notifier)":errorcluster)  [unwired: 1 in, 2 out]
  n1307 = local write "error out (LSI218)"(w31) -> ()
